vi "Advanced Cut - Main.vi"   [LabVIEW 2016] (continued)
"Rz Accel-in-Head", "Global Trigger", "", "", ""]; "Parameter Impuls Series"."Gain" format="%.1f"; "Parameter Impuls Series"."Offset" format="%.1f"})   [LabVIEW 2016]
uses:
  core/type-defs/TD_Statemachine-Data.ctl
  <userlib>/Import Export/Excel/Excel.lvclass
  core/type-defs/TD_Time Series.ctl
  core/type-defs/TD_Impulse Parameter.ctl
  Type Definitions/Advanced Cut - Forward Auto Cut.ctl
  Type Definitions/Advanced Cut - Reverse Auto Cut.ctl
  Type Definitions/Advanced Cut - Equal Auto Cut.ctl
  Type Definitions/Advanced Cut States.ctl
  UI/Listbox Class/MCListbox with Checkboxes.lvclass
  core/core.lvlib
panel:
  in  "Check All":bool
  in  "Snippet Table":i32(listbox)
  in  "Auto Cut Options":enum32{"->", "<-", "=="}(tab)
  in  "Auto Cut (Forward)":T1={"Start Time (s)"=0.0, "# Epochs"=10, "Epoch Duration (s)"=90.0} {"Epoch Duration (s)" min=0.0 step=1.0; "Start Time (s)" min=0.0 step=1.0}
  in  "Auto Cut (Reverse)":T2={"End Time (s)"=0.0, "# Epochs"=10, "Epoch Duration (s)"=90.0} {"Epoch Duration (s)" min=0.0 step=1.0; "End Time (s)" min=0.0 step=1.0}
  in  "Auto Cut (Equal)":T3={"Start Time (s)"=0.0, "End Time (s)"=90.0, "# Epochs"=10} {"End Time (s)" min=0.0 step=1.0; "Start Time (s)" min=0.0 step=1.0}
  in  "btn_ClearTable":bool
  in  "btn_AutoSnippet":bool
  in  "bool_KeepImpulses?":bool=TRUE
  in  "btn_DoCut":bool
  in  "Snippet File Suffix":string="_epoch"
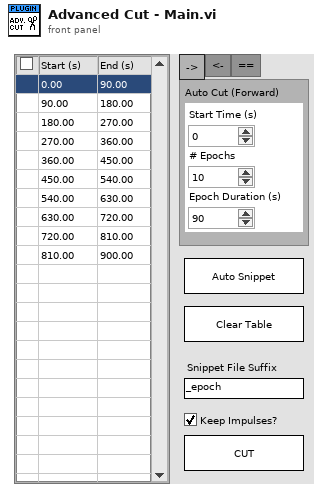
[diagram p1: front panel]
types:
  T1 = typedef "Advanced Cut - Forward Auto Cut.ctl" = cluster{"Start Time (s)":dbl, "# Epochs":u32, "Epoch Duration (s)":dbl}
  T2 = typedef "Advanced Cut - Reverse Auto Cut.ctl" = cluster{"End Time (s)":dbl, "# Epochs":u32, "Epoch Duration (s)":dbl}
  T3 = typedef "Advanced Cut - Equal Auto Cut.ctl" = cluster{"Start Time (s)":dbl, "End Time (s)":dbl, "# Epochs":u32}
  T4 = typedef "core.lvlib/TD_Statemachine-Data.ctl" = cluster{"Impulse Positions":cluster{"Start":i32, "End":i32, "Impulse Plane":enum16{"Other", "Yaw", "Pitch", "Roll", "LARP", "RALP"}, "Impulse Direction +ve?":bool, "Time offset":i32, "Amplitude offset":dbl}[], "No. Imp":i32, "Parameter Time Series":T5, "Parameter Impuls Series":T6, "Experiment Parameters":cluster{"Freq":dbl, "Vel":i32, "Acc":i32, "Stimulus":string}, "Autosort File":refnum<file>, "Data File":cluster{"Data Channels":dbl[][], "Sample Rate":i32, "Channel List":string[]}, "Experiment data path":path, "Image data path":path, "LVS data path":path, "Raw copy path":path, "filename":string, "desaccading parameters":cluster{"Tolerance":i32, "Acc Range":dbl, "Sample Rate":i32, "Impulse Plane 2":enum16{"Other", "Yaw", "Pitch", "Roll", "LARP", "RALP"}, "Impulse dir":bool}, "Experiment Parameters 2":cluster{"Subject":string, "Strain":string, "Rotation plane":string, "Experimenter":string, "Trial":dbl, "Time":dbl}, "Excel":cluster{"Excel._Application":refnum<k7>, "Use Excel":bool, "Worksheet SINE":refnum<k7>, "Row SINE":i32, "Worksheet TRANS":refnum<k7>, "Row TRANS":i32}, "Session Config File":refnum<file>, "Autosort Parameter Set":i32, "EMA Version":string, "desacc ":cluster{"Threshold 1 [Acc]":dbl, "Threshold 2 [% of TH1]":i32, "tolerance":i32, "Search WD ":dbl, " always use TH2":bool, "Range":dbl, "Max time":dbl, "Min time":dbl, "Velocity Threshold":i32}, "Cycle Nr for Saccades":cluster{"POS":i32, "NEG":i32}, "calibration name":string, "Excel":refnum<class "Excel.lvclass">}
  T5 = typedef "core.lvlib/TD_Time Series.ctl" = cluster{"time offset":dbl, "Offset":dbl, "Gain":dbl, "inverse":bool, "filter data":bool, "dots":bool, "interpolate":bool, "List 1":u16, "Color Box":u32, "Boolean":bool}[]
  T6 = typedef "core.lvlib/TD_Impulse Parameter.ctl" = cluster{"Color":u32, "Visible":bool, "Channel":u16, "Invert":bool, "Desaccade":bool, "Offset":dbl, "Gain":dbl}[]
  T7 = typedef "Advanced Cut States.ctl" = enum16{"Initialise", "Quit", "DO Refresh Snippet Table", "DO Auto Snippet", "DO Clear Snippets", "DO Cut"}
  T8 = cluster{"left":i16, "top":i16, "right":i16, "bottom":i16}
  T9 = typedef "LVPoint32TypeDef.ctl" = cluster{"Horizontal":i32, "Vertical":i32}
  T10 = typedef "LVRowAndColumnTypeDef.ctl" = cluster{"Row":i32, "Column":i32}
  T11 = typedef "eventvkey.ctl" = enum16{"ASCII", "Enter", "Return", "Shift", "Ctrl", "Alt", "Cmd", "Opt", "Caps", "NumLock", "Clear", "Break", "Up", "Down", "Left", "Right", "Insert", "Delete", "Home", "End", "PageUp", "PageDown", "Escape", "Help", "Pause", "ScrollLock", "F1", "F2", "F3", "F4", "F5", "F6", "F7", "F8", "F9", "F10", "F11", "F12", "F13", "F14", "F15", "F16", "F17", "F18", "F19", "F20", "F21", "F22", "F23", "F24", "Play", "VolumeUp", "VolumeDown", "Mute", "Two Byte Char"}
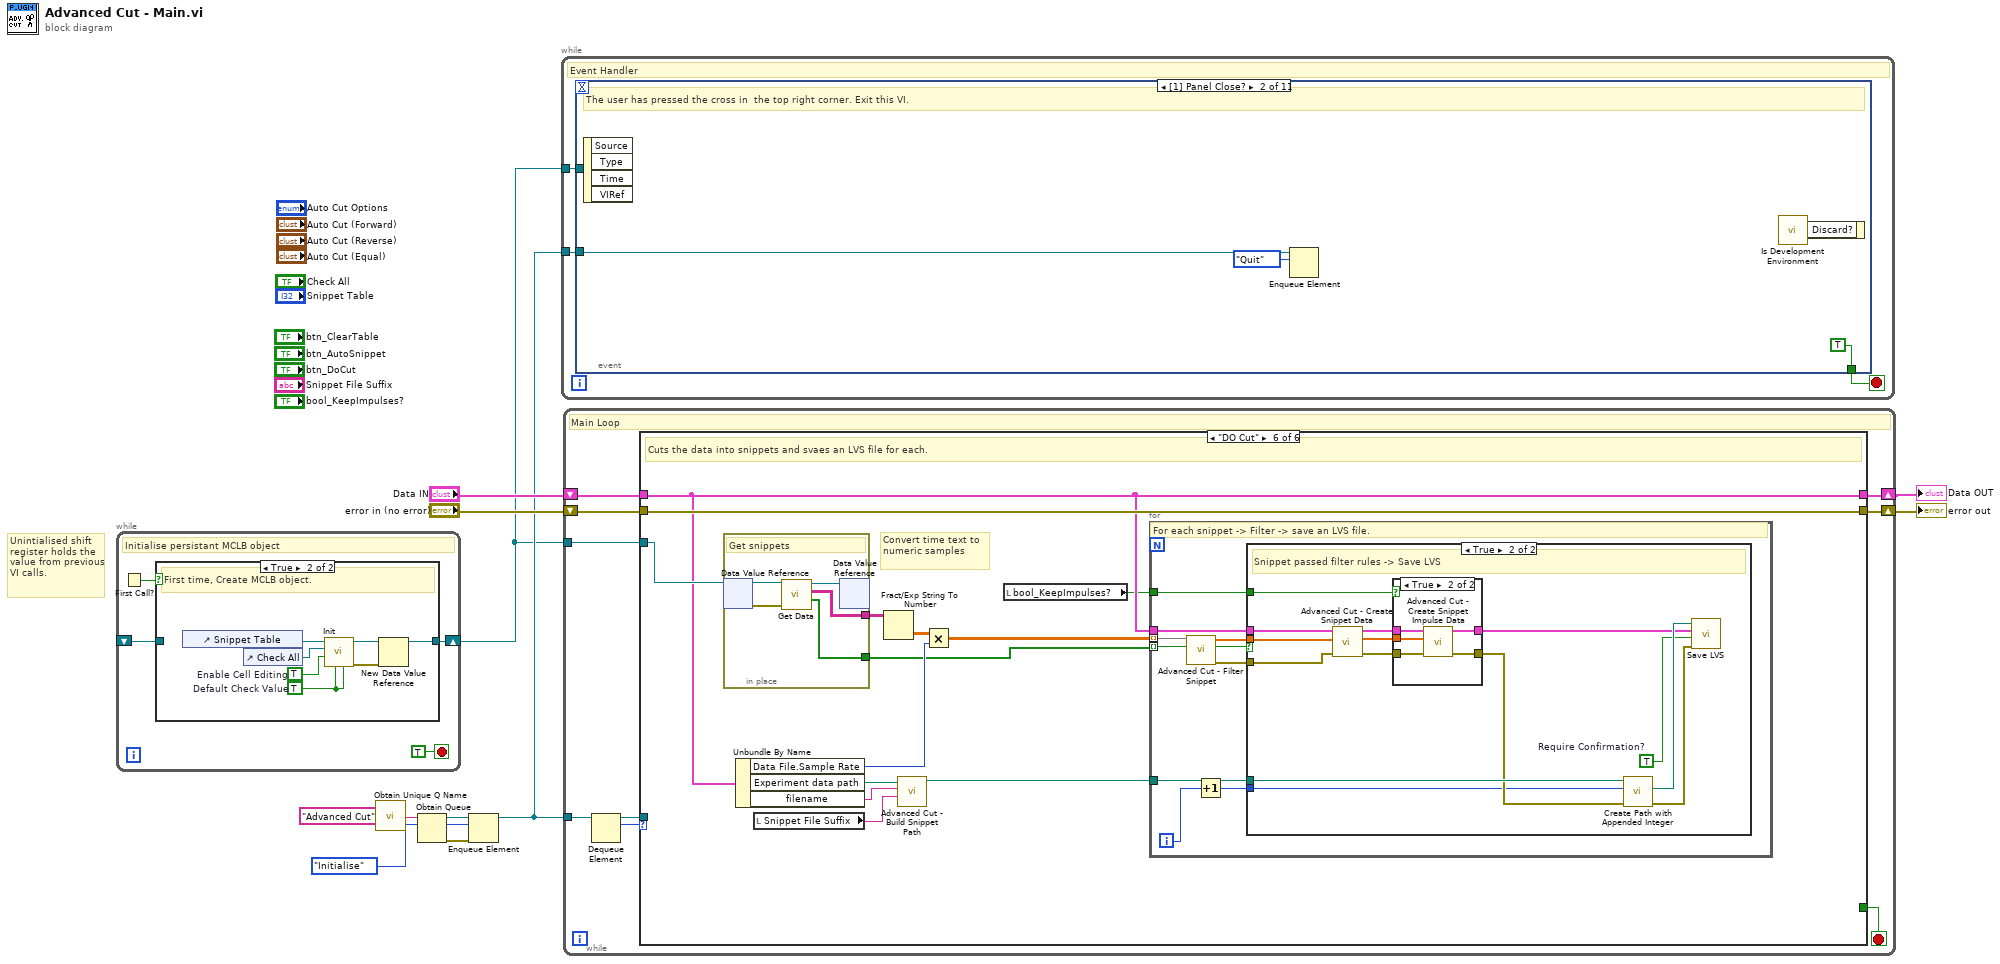
[diagram p0: block diagram]
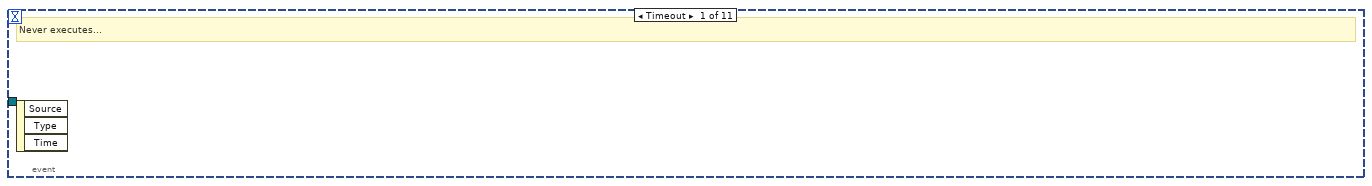
[diagram p3: hidden frame]
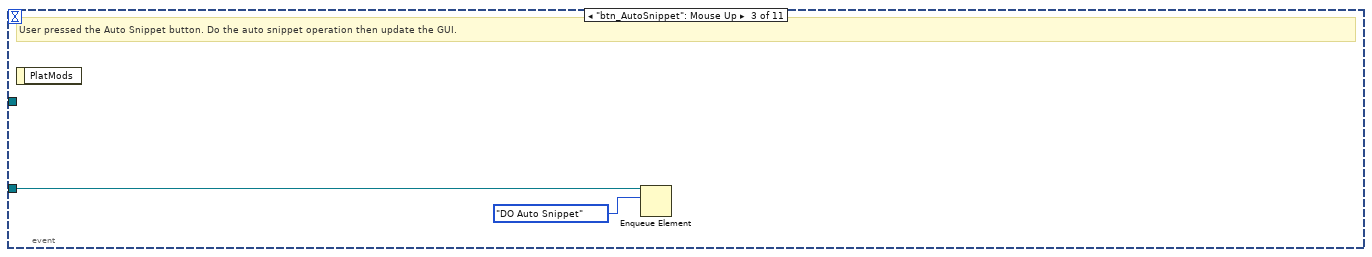
[diagram p4: hidden frame]
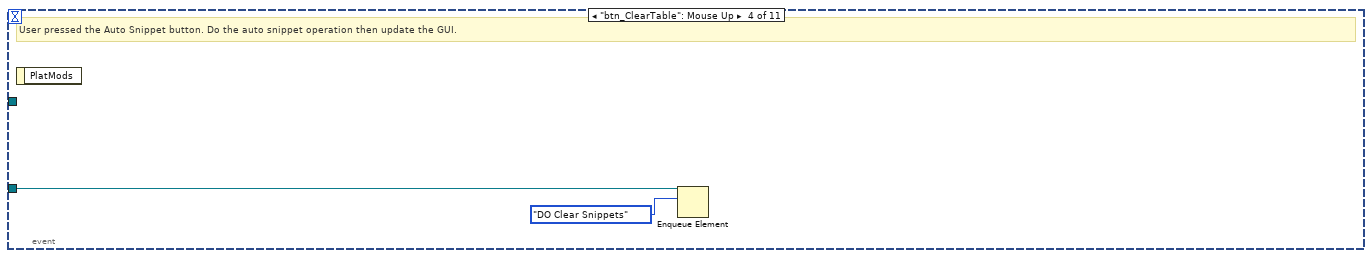
[diagram p5: hidden frame]
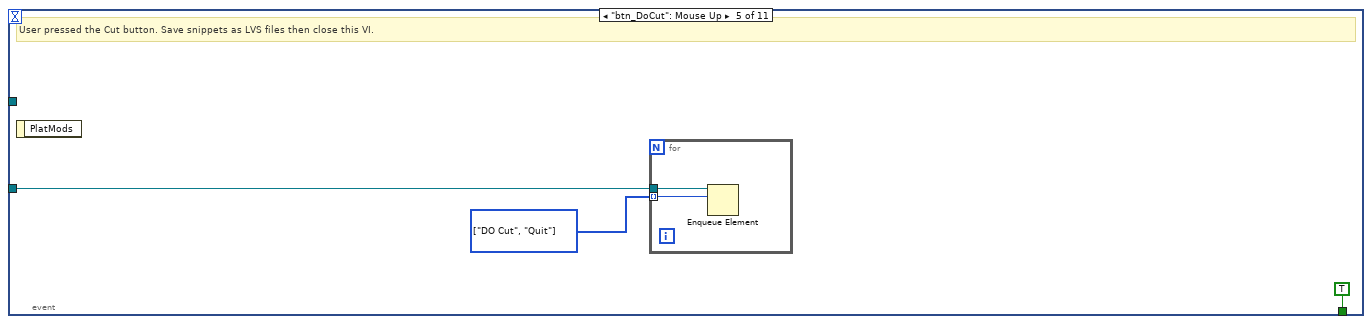
[diagram p6: hidden frame]
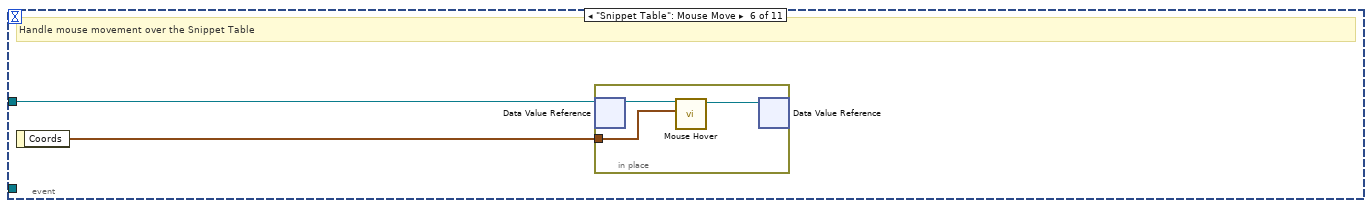
[diagram p7: hidden frame]
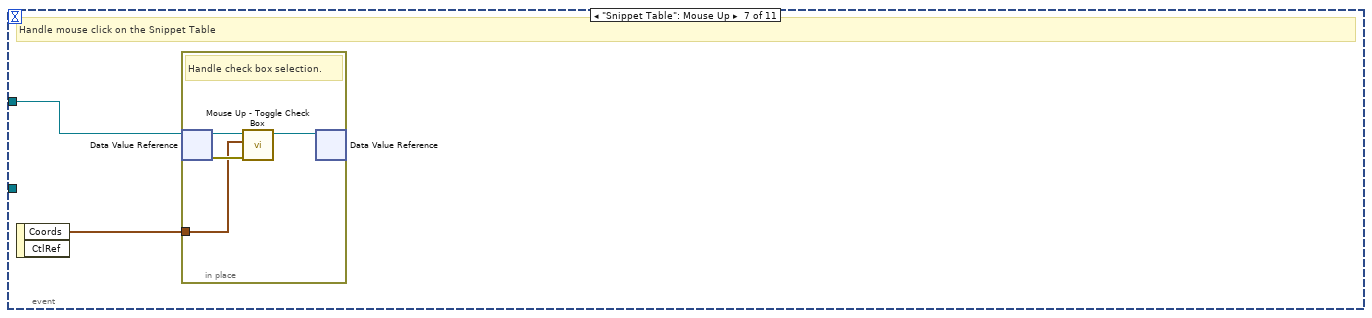
[diagram p8: hidden frame]
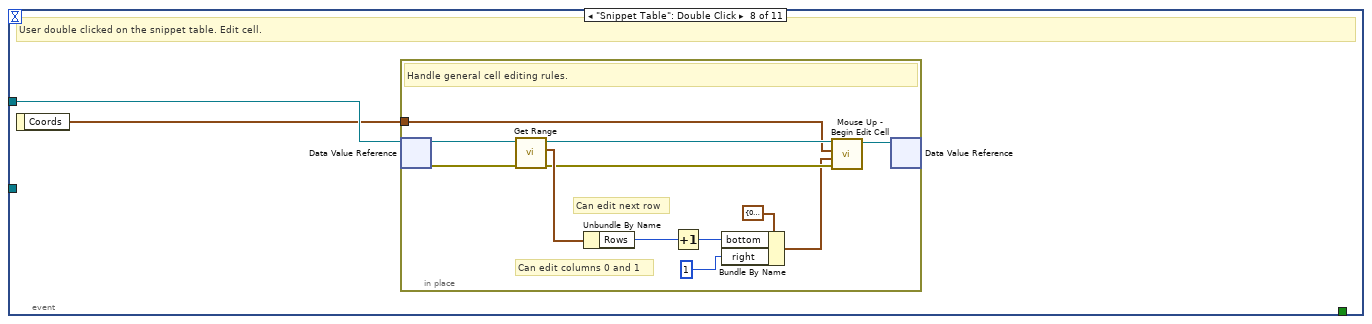
[diagram p9: hidden frame]
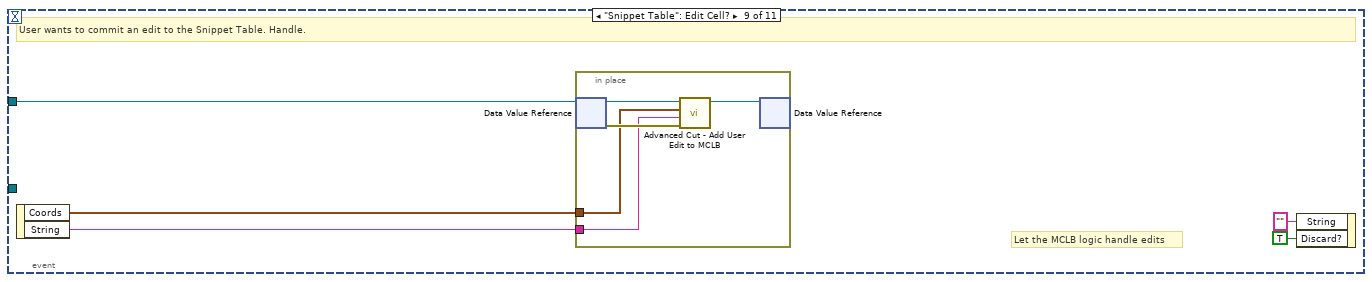
[diagram p10: hidden frame]
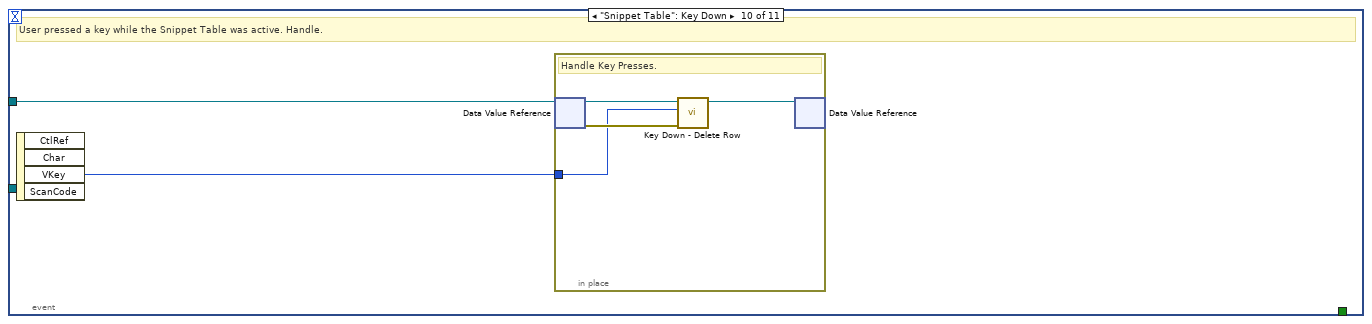
[diagram p11: hidden frame]
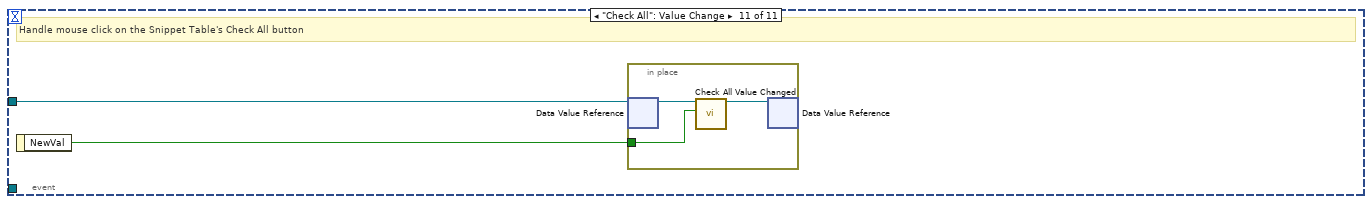
[diagram p12: hidden frame]
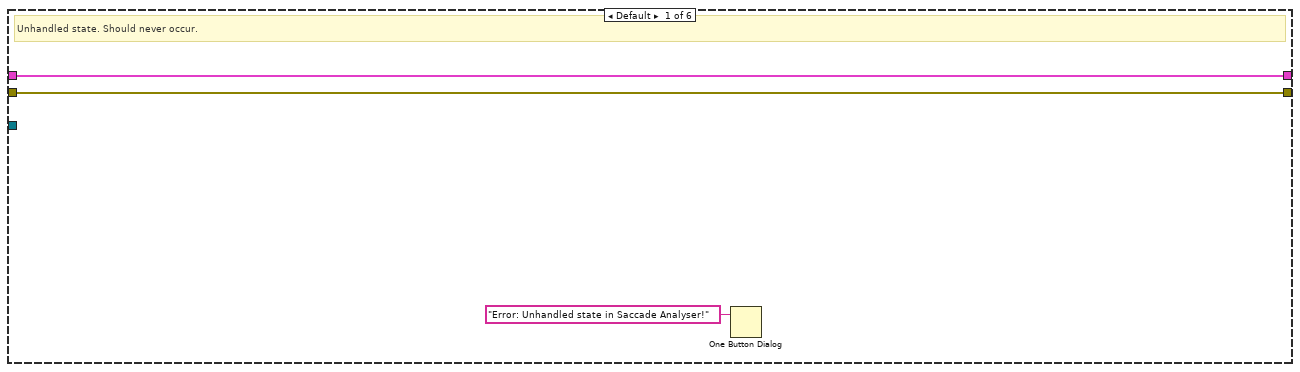
[diagram p13: hidden frame]
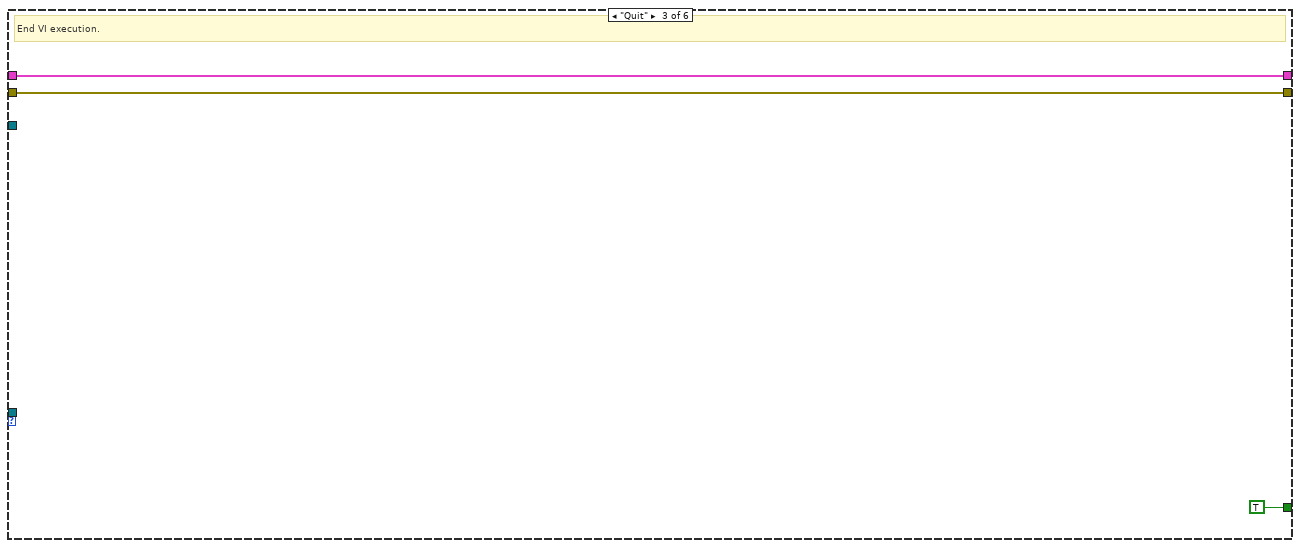
[diagram p15: hidden frame]
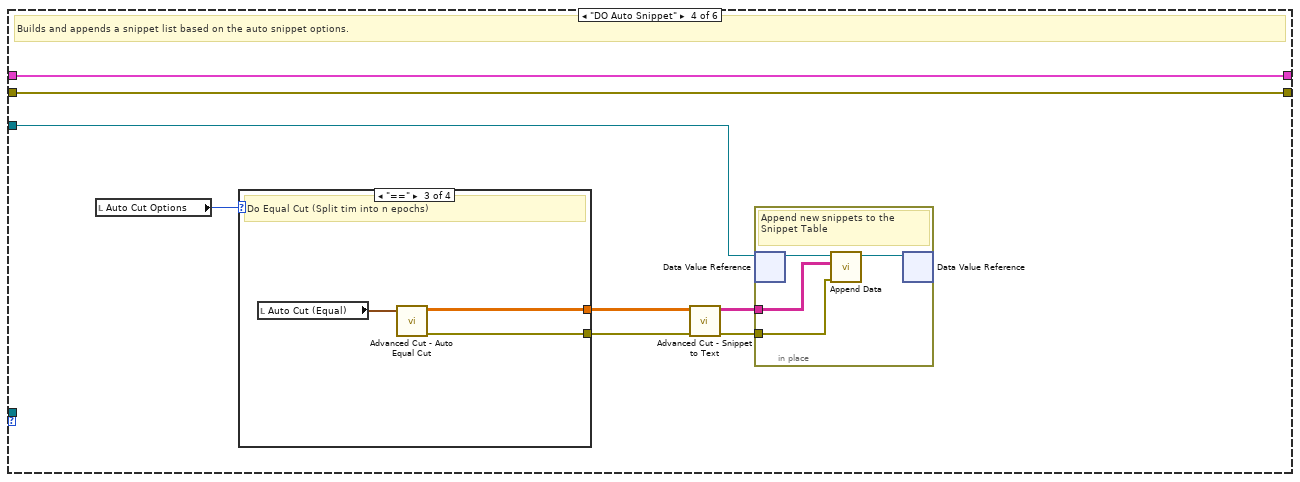
[diagram p16: hidden frame]
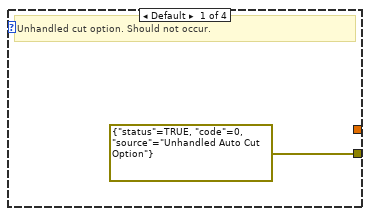
[diagram p17: hidden frame]
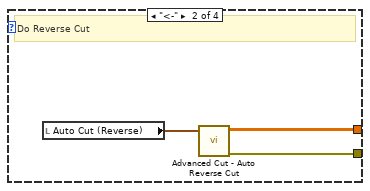
[diagram p18: hidden frame]
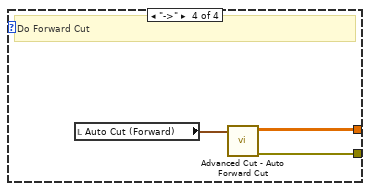
[diagram p19: hidden frame]
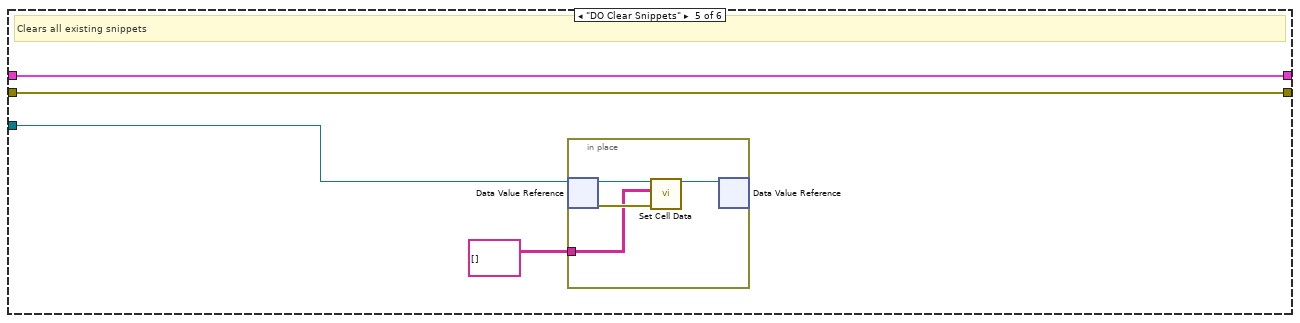
[diagram p20: hidden frame]
diagram:
  w3 = Advanced_Cut_States."Initialise" ("Advanced Cut States")
  # "Unintialised shift register holds the value from previous VI calls."
  n1 = while {
    shift-right: [w13] -> w1
    shift-left: _ -> [w12]
    stop <- TRUE stop-if-true
    # "Initialise persistant MCLB object"
    n2 = First Call?() -> (First Call?: T/F=w14:bool)
    n3 = case shown="True" w14 {
      tunnel: [w16 w17] -> w13
      tunnel: w12 -> [w16 _]
      frame False {
        # "Not first time, reuse existing object."
      }
      frame True {
        w23 = TRUE  # Enable Cell Editing
        w22 = TRUE  # Default Check Value
        # "First time, Create MCLB object."
        n4 = control-ref of="Snippet Table"() -> (w18:refnum<vi>)
        n5 = control-ref of="Check All"() -> (w19:refnum<vi>)
        n6 = call "Init.vi"("Default Check Value (F)"=w22, "Check Value (F)"=w22, "Enable Cell Editing (F)"=w23, "Check All"=w19, "Multicolumn Listbox"=w18) -> ("error out"=w20:errorcluster, "MCListbox with Checkboxes.lvclass"=w21:refnum<class "MCListbox with Checkboxes.lvclass">)  [unwired: 5 in]
        n7 = New Data Value Reference(data value=w21, error in=w20) -> (data value reference=w17:refnum<data-value>)  [unwired: 1 out]
      }
    }
  }
  n8 = call <userlib>:"Obtain Unique Q Name.vi"("Queue"="Advanced Cut") -> ("Q Name"=w4:string)  [unwired: 4 in]
  n9 = Obtain Queue(name (unnamed)=w4, element data type=w3) -> (queue out=w6:refnum<queue>, error out=w7:errorcluster)  [unwired: 3 in, 1 out]
  n10 = Enqueue Element(queue=w6, element=w3, error in (no error)=w7) -> (queue out=w2:refnum<queue>)  [unwired: 1 in, 2 out]
  n11 = while {
    tunnel: w2 -> [w25]
    tunnel: w1 -> [w24]
    stop <- w26 stop-if-true
    # "Event Handler"
    n12 = event shown="[1] Panel Close?" {
      selector: _ -> [_ _ _ _ _ _ _ _ _ _ _]
      dyn-events: _ -> [_ _ _ _ _ _ _ _ _ _ _]
      timeout: _ -> [_ _ _ _ _ _ _ _ _ _ _]
      tunnel: [_ TRUE _ _ TRUE _ _ _ _ _ _] -> w26
      tunnel: w25 -> [_ w28 w32 w33 w37 _ _ _ _ _ _]
      tunnel: w24 -> [_ _ _ _ _ w40 w46 w52 w69 w76 w82]
      event Timeout {
        # "Never executes..."
        n13 = event-data() -> ()  [unwired: 1 in, 3 out]
      }
      event Panel Close? {
        # "The user has pressed the cross in  the top right corner. Exit this VI."
        n14 = event-data() -> ()  [unwired: 1 in, 4 out]
        n15 = Enqueue Element(queue=w28, element=Advanced_Cut_States."Quit") -> ()  [unwired: 2 in, 3 out]
        n16 = call <userlib>:"Is Development Environment.vi"() -> ("exe?"=w30:bool)  [unwired: 5 in]
        n17 = event-data("Discard?"=w30) -> ()  [unwired: 1 in, 1 out]
      }
      event "btn_AutoSnippet": Mouse Up {
        # "User pressed the Auto Snippet button. Do the auto snippet operation then update the GUI."
        n18 = event-data() -> ()  [unwired: 1 in, 1 out]
        n19 = Enqueue Element(queue=w32, element=Advanced_Cut_States."DO Auto Snippet" ("Advanced Cut States")) -> ()  [unwired: 2 in, 3 out]
      }
      event "btn_ClearTable": Mouse Up {
        # "User pressed the Auto Snippet button. Do the auto snippet operation then update the GUI."
        n20 = event-data() -> ()  [unwired: 1 in, 1 out]
        n21 = Enqueue Element(queue=w33, element=Advanced_Cut_States."DO Clear Snippets" ("Advanced Cut States")) -> ()  [unwired: 2 in, 3 out]
      }
      event "btn_DoCut": Mouse Up {
        w36 = T7[] [enum."DO Cut", enum."Quit"] items=["Initialise", "Quit", "DO Refresh Snippet Table", "DO Auto Snippet", "DO Clear Snippets", "DO Cut"] ("element")
        # "User pressed the Cut button. Save snippets as LVS files then close this VI."
        n22 = event-data() -> ()  [unwired: 1 in, 1 out]
        n23 = for {
          tunnel: w37 -> [w39]
          tunnel: w36 -> [w38] mode=indexing
          n24 = Enqueue Element(queue=w39, element=w38) -> ()  [unwired: 2 in, 3 out]
        }
      }
      event "Snippet Table": Mouse Move {
        # "Handle mouse movement over the Snippet Table"
        n25 = event-data() -> ("Coords"=w41:T9)  [unwired: 1 in]
        n26 = in-place {
          in-place-border: w41 -> [w44]
          n27 = in-place-dvr #1(w40) -> (w43:refnum<class "MCListbox with Checkboxes.lvclass">)  [unwired: 1 out]
          n28 = call "Mouse Hover.vi"("Coords"=w44, "MCListbox with Checkboxes in"=w43) -> ("MCListbox with Checkboxes out"=w42:refnum<class "MCListbox with Checkboxes.lvclass">)  [unwired: 8 in, 1 out]
          n29 = in-place-dvr #1(w42) -> ()  [unwired: 2 out]
        }
      }
      event "Snippet Table": Mouse Up {
        # "Handle mouse click on the Snippet Table"
        n30 = event-data() -> ("Coords"=w45:T9)  [unwired: 1 in, 1 out]
        n31 = in-place {
          in-place-border: w45 -> [w48]
          # "Handle check box selection."
          n32 = in-place-dvr #2(w46) -> (w50:refnum<class "MCListbox with Checkboxes.lvclass">, w49:errorcluster)
          n33 = call "Mouse Up - Toggle Check Box.vi"("error in (no error)"=w49, "Coords"=w48, "MCListbox with Checkboxes in"=w50) -> ("MCListbox with Checkboxes out"=w47:refnum<class "MCListbox with Checkboxes.lvclass">)  [unwired: 6 in, 2 out]
          n34 = in-place-dvr #2(w47) -> ()  [unwired: 2 out]
        }
      }
      event "Snippet Table": Double Click {
        # "User double clicked on the snippet table. Edit cell."
        n35 = event-data() -> ("Coords"=w51:T9)  [unwired: 1 in]
        n36 = in-place {
          in-place-border: w51 -> [w56]
          # "Can edit columns 0 and 1"
          # "Can edit next row"
          # "Handle general cell editing rules."
          n37 = in-place-dvr #3(w52) -> (w54:refnum<class "MCListbox with Checkboxes.lvclass">, w53:errorcluster)
          n38 = call "Get Range.vi"("error in (no error)"=w53, "MCListbox with Checkboxes in"=w54) -> ("error out"=w58:errorcluster, "Range"=w63:cluster{"Rows":i32, "Columns":i32}, "MCListbox with Checkboxes out"=w59:refnum<class "MCListbox with Checkboxes.lvclass">)  [unwired: 7 in]
          n39 = Unbundle By Name(w63) -> ("Rows"=w62:i32)
          n40 = Increment(x=w62) -> (x+1=w61:i32)
          n41 = Bundle By Name(cluster=T8 {"left"=0, "top"=0, "right"=0, "bottom"=0} ("Valid Region"), "bottom"=w61, "right"=i16 1) -> (w55:T8)
          n42 = call "Mouse Up - Begin Edit Cell.vi"("error in (no error)"=w58, "Valid Region"=w55, "Coords"=w56, "MCListbox with Checkboxes in"=w59) -> ("MCListbox with Checkboxes out"=w57:refnum<class "MCListbox with Checkboxes.lvclass">)  [unwired: 5 in, 2 out]
          n43 = in-place-dvr #3(w57) -> ()  [unwired: 2 out]
        }
      }
      event "Snippet Table": Edit Cell? {
        # "Let the MCLB logic handle edits"
        # "User wants to commit an edit to the Snippet Table. Handle."
        n44 = event-data() -> ("Coords"=w68:T10, "String"=w67:string)  [unwired: 1 in]
        n45 = in-place {
          in-place-border: w68 -> [w72]
          in-place-border: w67 -> [w71]
          n46 = in-place-dvr #4(w69) -> (w74:refnum<class "MCListbox with Checkboxes.lvclass">, w73:errorcluster)
          n47 = call "Advanced Cut - Add User Edit to MCLB.vi"("error in (no error)"=w73, "Edit Value"=w71, "RowAndCollumn"=w72, "MCListbox with Checkboxes in"=w74) -> ("MCListbox with Checkboxes out"=w70:refnum<class "MCListbox with Checkboxes.lvclass">)  [unwired: 5 in, 2 out]
          n48 = in-place-dvr #4(w70) -> ()  [unwired: 2 out]
        }
        n49 = event-data("String"="", "Discard?"=TRUE) -> ()  [unwired: 1 in, 1 out]
      }
      event "Snippet Table": Key Down {
        # "User pressed a key while the Snippet Table was active. Handle."
        n50 = event-data() -> ("VKey"=w75:T11)  [unwired: 1 in, 3 out]
        n51 = in-place {
          in-place-border: w75 -> [w78]
          # "Handle Key Presses."
          n52 = in-place-dvr #5(w76) -> (w80:refnum<class "MCListbox with Checkboxes.lvclass">, w79:errorcluster)
          n53 = call "Key Down - Delete Row.vi"("error in (no error)"=w79, "Key Pressed in"=w78, "MCListbox with Checkboxes in"=w80) -> ("MCListbox with Checkboxes out"=w77:refnum<class "MCListbox with Checkboxes.lvclass">)  [unwired: 6 in, 2 out]
          n54 = in-place-dvr #5(w77) -> ()  [unwired: 2 out]
        }
      }
      event "Check All": Value Change {
        # "Handle mouse click on the Snippet Table's Check All button"
        n55 = event-data() -> ("NewVal"=w81:bool)  [unwired: 1 in]
        n56 = in-place {
          in-place-border: w81 -> [w83]
          n57 = in-place-dvr #6(w82) -> (w85:refnum<class "MCListbox with Checkboxes.lvclass">)  [unwired: 1 out]
          n58 = call "Check All Value Changed.vi"("New Value"=w83, "MCListbox with Checkboxes in"=w85) -> ("MCListbox with Checkboxes out"=w84:refnum<class "MCListbox with Checkboxes.lvclass">)  [unwired: 8 in, 1 out]
          n59 = in-place-dvr #6(w84) -> ()  [unwired: 2 out]
        }
      }
    }
  }
  n60 = while {
    shift-right: [w91] -> w9
    shift-left: "Data IN" -> [w92]
    shift-right: [w89] -> w8
    shift-left: "error in (no error)" -> [w90]
    tunnel: w2 -> [w94]
    tunnel: w1 -> [w86]
    stop <- w88 stop-if-true
    # "Main Loop"
    n61 = Dequeue Element(queue=w94) -> (queue out=w87:refnum<queue>, element=w93:T7)  [unwired: 2 in, 2 out]
    n62 = case shown="\"DO Cut\"" w93 {
      tunnel: w92 -> [w96 w98 w102 w109 w127 w143]
      tunnel: [w96 w98 w102 w109 w127 w143] -> w91
      tunnel: w90 -> [w95 w99 w101 w110 w128 w145]
      tunnel: [w95 w99 w101 w110 w128 w145] -> w89
      tunnel: [_ _ TRUE _ _ _] -> w88
      tunnel: w87 -> [_ _ _ _ _ _]
      tunnel: w86 -> [_ _ _ w108 w126 w144]
      frame Default {
        # "Unhandled state. Should never occur."
        n63 = One Button Dialog(message="Error: Unhandled state in Saccade Analyser!") -> ()  [unwired: 1 in, 1 out]
      }
      frame "Initialise" {
        # "Configure VI for execution."
      }
      frame "Quit" {
        # "End VI execution."
      }
      frame "DO Auto Snippet" {
        # "Builds and appends a snippet list based on the auto snippet options."
        n64 = local read "Auto Cut Options"() -> (w103:enum32{"->", "<-", "=="})
        n65 = case shown="\"==\"" w103 {
          tunnel: [_ w113 w116 w120] -> w107
          tunnel: [errorcluster {"status"=TRUE, "code"=0, "source"="Unhandled Auto Cut Option"} ("error out") w112 w115 w118] -> w105
          frame Default {
            # "Unhandled cut option. Should not occur."
          }
          frame "<-" {
            # "Do Reverse Cut"
            n66 = local read "Auto Cut (Reverse)"() -> (w114:T2)
            n67 = call "Advanced Cut - Auto Reverse Cut.vi"("Auto Cut (Reverse)"=w114) -> ("error out"=w112:errorcluster, "Snippets"=w113:dbl[][])  [unwired: 9 in]
          }
          frame "==" {
            # "Do Equal Cut (Split tim into n epochs)"
            n68 = local read "Auto Cut (Equal)"() -> (w117:T3)
            n69 = call "Advanced Cut - Auto Equal Cut.vi"("Auto Cut (Equal)"=w117) -> ("error out"=w115:errorcluster, "Snippets"=w116:dbl[][])  [unwired: 9 in]
          }
          frame "->" {
            # "Do Forward Cut"
            n70 = local read "Auto Cut (Forward)"() -> (w119:T1)
            n71 = call "Advanced Cut - Auto Forward Cut.vi"("Auto Cut (Forward)"=w119) -> ("error out"=w118:errorcluster, "Snippets"=w120:dbl[][])  [unwired: 9 in]
          }
        }
        n72 = call "Advanced Cut - Snippet to Text.vi"("error in (no error)"=w105, "Numeric Snippets"=w107) -> ("error out"=w104:errorcluster, "String Snippets"=w106:string[][])  [unwired: 8 in]
        n73 = in-place {
          in-place-border: w106 -> [w122]
          in-place-border: w104 -> [w121]
          # "Append new snippets to the Snippet Table"
          n74 = in-place-dvr #7(w108) -> (w124:refnum<class "MCListbox with Checkboxes.lvclass">)  [unwired: 1 out]
          n75 = call "Append Data.vi"("error in (no error)"=w121, "Cell Data"=w122, "MCListbox with Checkboxes in"=w124) -> ("MCListbox with Checkboxes out"=w123:refnum<class "MCListbox with Checkboxes.lvclass">)  [unwired: 7 in, 1 out]
          n76 = in-place-dvr #7(w123) -> ()  [unwired: 2 out]
        }
      }
      frame "DO Clear Snippets" {
        # "Clears all existing snippets"
        n77 = in-place {
          in-place-border: string[][] [] ("Cell Data") -> [w129]
          n78 = in-place-dvr #8(w126) -> (w132:refnum<class "MCListbox with Checkboxes.lvclass">, w130:errorcluster)
          n79 = call "Set Cell Data.vi"("error in (no error)"=w130, "Cell Data"=w129, "MCListbox with Checkboxes in"=w132) -> ("MCListbox with Checkboxes out"=w131:refnum<class "MCListbox with Checkboxes.lvclass">)  [unwired: 7 in, 1 out]
          n80 = in-place-dvr #8(w131) -> ()  [unwired: 2 out]
        }
      }
      frame "DO Cut" {
        # "Convert time text to numeric samples"
        # "Cuts the data into snippets and svaes an LVS file for each."
        n81 = in-place {
          in-place-border: [w147] -> w142
          in-place-border: [w146] -> w133
          # "Get snippets"
          n82 = in-place-dvr #9(w144) -> (w150:refnum<class "MCListbox with Checkboxes.lvclass">, w149:errorcluster)
          n83 = call "Get Data.vi"("error in (no error)"=w149, "MCListbox with Checkboxes in"=w150) -> ("Check Data"=w146:bool[], "Cell Data"=w147:string[][], "MCListbox with Checkboxes out"=w148:refnum<class "MCListbox with Checkboxes.lvclass">)  [unwired: 6 in, 1 out]
          n84 = in-place-dvr #9(w148) -> ()  [unwired: 2 out]
        }
        n85 = Unbundle By Name(w143) -> ("Data File.Sample Rate"=w135:i32, "Experiment data path"=w140:path, "filename"=w139:string)
        n86 = local read "Snippet File Suffix"() -> (w138:string)
        n87 = Fract/Exp String To Number(string=w142) -> (number=w141:dbl[][])  [unwired: 3 in, 1 out]
        n88 = call "Advanced Cut - Build Snippet Path.vi"("Snippet Suffix"=w138, "Original File Name"=w139, "Destination Directory"=w140) -> ("Snippet Path"=w137:path)  [unwired: 7 in, 1 out]
        n89 = Multiply(x=w141, y=w135) -> (x*y=w134:dbl[][])
        n90 = local read "bool_KeepImpulses?"() -> (w136:bool)
        n91 = for {
          tunnel: w143 -> [w159]
          tunnel: w137 -> [w160]
          tunnel: w134 -> [w157] mode=indexing
          tunnel: w136 -> [w158]
          tunnel: w133 -> [w154] mode=indexing
          i -> [w152]
          # "For each snippet -> Filter -> save an LVS file."
          n92 = call "Advanced Cut - Filter Snippet.vi"("Include?"=w154, "Snippet in"=w157) -> ("error out"=w155:errorcluster, "Pass?"=w153:bool, "Snippet out"=w156:dbl[])  [unwired: 7 in]
          n93 = Increment(x=w152) -> (x+1=w151:i32)
          n94 = case shown="True" w153 {
            tunnel: w160 -> [_ w167]
            tunnel: w159 -> [_ w174]
            tunnel: w158 -> [_ w170]
            tunnel: w156 -> [_ w169]
            tunnel: w155 -> [_ w168]
            tunnel: w151 -> [_ w163]
            frame False {
              # "Snippet did not pass filter rules -> Skip."
            }
            frame True {
              w162 = TRUE  # Require Confirmation?
              # "Snippet passed filter rules -> Save LVS"
              n95 = call "Advanced Cut - Create Snippet Data.vi"("error in (no error)"=w168, "Snippet Domain in (samples)"=w169, "Data IN"=w174) -> ("error out"=w171:errorcluster, "Snippet Domain out (samples)"=w172:dbl[], "Data OUT"=w173:T4)  [unwired: 6 in]
              n96 = case shown="True" w170 {
                tunnel: w173 -> [w179 w184]
                tunnel: w172 -> [w178 w183]
                tunnel: w171 -> [w176 w182]
                tunnel: [w177 w181] -> w161
                tunnel: [w175 w180] -> w166
                frame False {
                  n97 = call "Advanced Cut - Remove Snippet Impulse Data.vi"("error in (no error)"=w176, "Snippet Domain in (samples)"=w178, "Data IN"=w179) -> ("error out"=w175:errorcluster, "Data OUT"=w177:T4)  [unwired: 6 in, 1 out]
                }
                frame True {
                  n98 = call "Advanced Cut - Create Snippet Impulse Data.vi"("error in (no error)"=w182, "Snippet Domain in (samples)"=w183, "Data IN"=w184) -> ("error out"=w180:errorcluster, "Data OUT"=w181:T4)  [unwired: 6 in, 1 out]
                }
              }
              n99 = call "Create Path with Appended Integer.vi"("error in (no error)"=w166, "Path Number"=w163, "Base Path (in)"=w167) -> ("error out"=w164:errorcluster, "Numeric Appended Path"=w165:path)  [unwired: 6 in, 1 out]
              n100 = call "Save LVS.vi"("error in (no error)"=w164, "Require Confirmation? (F)"=w162, "LVS Data"=w161, "Path (in)"=w165) -> ()  [unwired: 6 in, 2 out]
            }
          }
        }
      }
    }
  }
  "Data OUT" <- w9
  "error out" <- w8
